vi "Configured Acquisition Trigger (Host)_20221229_Dual.vi"() -> ()   [LabVIEW 2021]
doc: "Use this VI as a template to design an application that acquires data using advanced triggering logic from the NI PXIe-5170R/5171R."
uses:
  Enums/Channel Numbers.ctl
  <vilib>/FPGAPlugInAG/PXIe-5172 (8CH - 410T)/niLvFpga_Open_PXIe-5172 (8CH - 410T).vi
  <vilib>/rvi/interface/common/dynamic/niFpgaDynamicAddResources.vi
  <vilib>/FPGAPlugInAG/Dynamic/niLvFpga_Close_Dynamic.vi
  <vilib>/rvi/interface/nirviOpenFPGA/nirviOpenFPGA.xnode
  FPGA Bitfiles/Multirecord Acquisition FPGA_20221228a_4.lvbitx
  <vilib>/rvi/interface/nirviCloseFPGA/nirviCloseFPGA.xnode
  Device Session/Device Session.lvclass
panel:
  out "Host Loop Count":i32
  out "Waveform Graph 1":T1(graph)
  out "TrigCfg Array":T2(array[cluster])
  out "TrigCount":u32[](array[numeric])
  in  "ResetTrig":bool=TRUE
  in  "Sliding Window Trigger":cluster{"Range":dbl, "StartCenter":dbl}[](array[cluster])=[{"Range"=2.01, "StartCenter"=0.0}, {"Range"=0.01, "StartCenter"=0.0}, {"Range"=5.0, "StartCenter"=0.0}, {"Range"=5.0, "StartCenter"=0.0}, {"Range"=5.0, "StartCenter"=0.0}, {"Range"=5.0, "StartCenter"=0.0}, {"Range"=5.0, "StartCenter"=0.0}, {"Range"=5.0, "StartCenter"=0.0}]
  out "actual sample rate":dbl format="%#_6p"
  in  "onboard sample clock rate":dbl(ring)=200000000.0 items=["250 MHz"=250000000.0, "200 MHz"=200000000.0, "150 MHz"=150000000.0]
  in  "impedance":enum8{"Default", "1 mega ohm", "50 ohm"}(ring)
  in  "vertical offset (V)":dbl format="%.2p"
  out "Waveform Graph 0":T1(graph)
  in  "mode":T3(ring)
  in  "decimation factor":u16=1
  in  "coupling":enum8{"Default", "DC", "AC"}(ring)
  in  "bandwidth":T4(ring)
  in  "pretrigger samples":u64=500
  in  "number of samples":u64=1000
  in  "RIO Device":tag="PXI2Slot3"
  in  "channel(s)":string="0,1,2,3,4,5,6,7"
  in  "vertical range (Vpp)":dbl=1.0 format="%.2p"
  out "error out":errorcluster
  in  "stop":bool
  # "RIO Device"
  # "Vertical Settings"
  # "Trigger Settings"
  # "Acquisition Settings"
  # "DSP"
  # "Clocking"
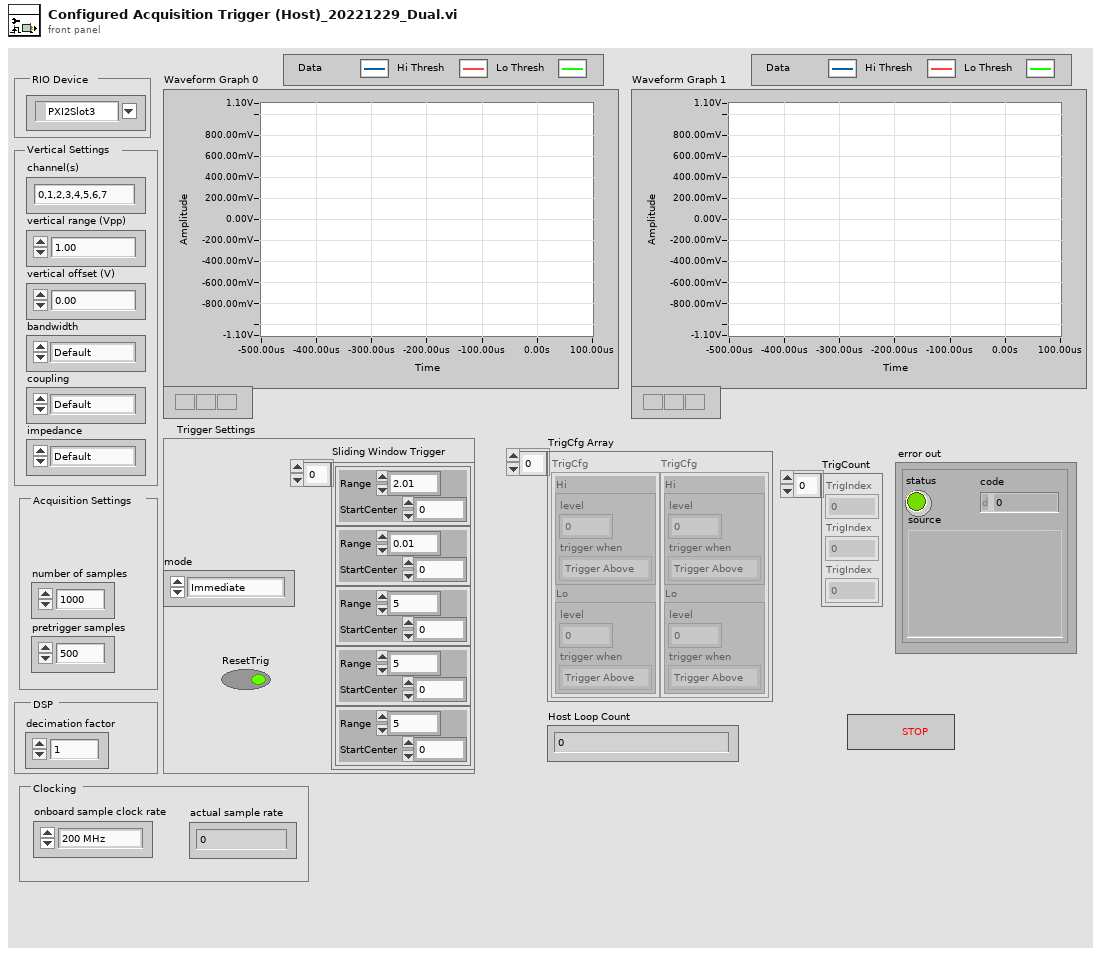
[diagram p1: front panel]
types:
  T1 = cluster{"relativeX":dbl, "sample rate":dbl, "data in":dbl[]}[]
  T2 = cluster{"Hi":cluster{"level":fxp<+/-,18,5>, "trigger when":enum8{"Trigger Above", "Trigger Below"}}, "Lo":cluster{"level":fxp<+/-,18,5>, "trigger when":enum8{"Trigger Above", "Trigger Below"}}}[]
  T3 = enum16{"Immediate", "A", "B", "OR", "AND", "A THEN B", "B THEN A", "High Resolution"}
  T4 = enum8{"Default", "Full Bandwidth", "Anti-alias Filter", "80 MHz FIR Filter", "40 MHz FIR Filter", "20 MHz FIR Filter"}
  T5 = typedef "Channel Numbers.ctl" = enum16{"0", "1", "2", "3", "4", "5", "6", "7"}
  T6 = typedef "niInstr Multirecord Acquisition v1 Host.lvclass/Scaling Coefficient.ctl" = cluster{"gain":dbl, "offset":dbl}
  T7 = typedef "ChannelWindowClust.ctl" = cluster{"HalfRange":fxp<+/-,18,5>, "StartCenter":fxp<+/-,18,5>}
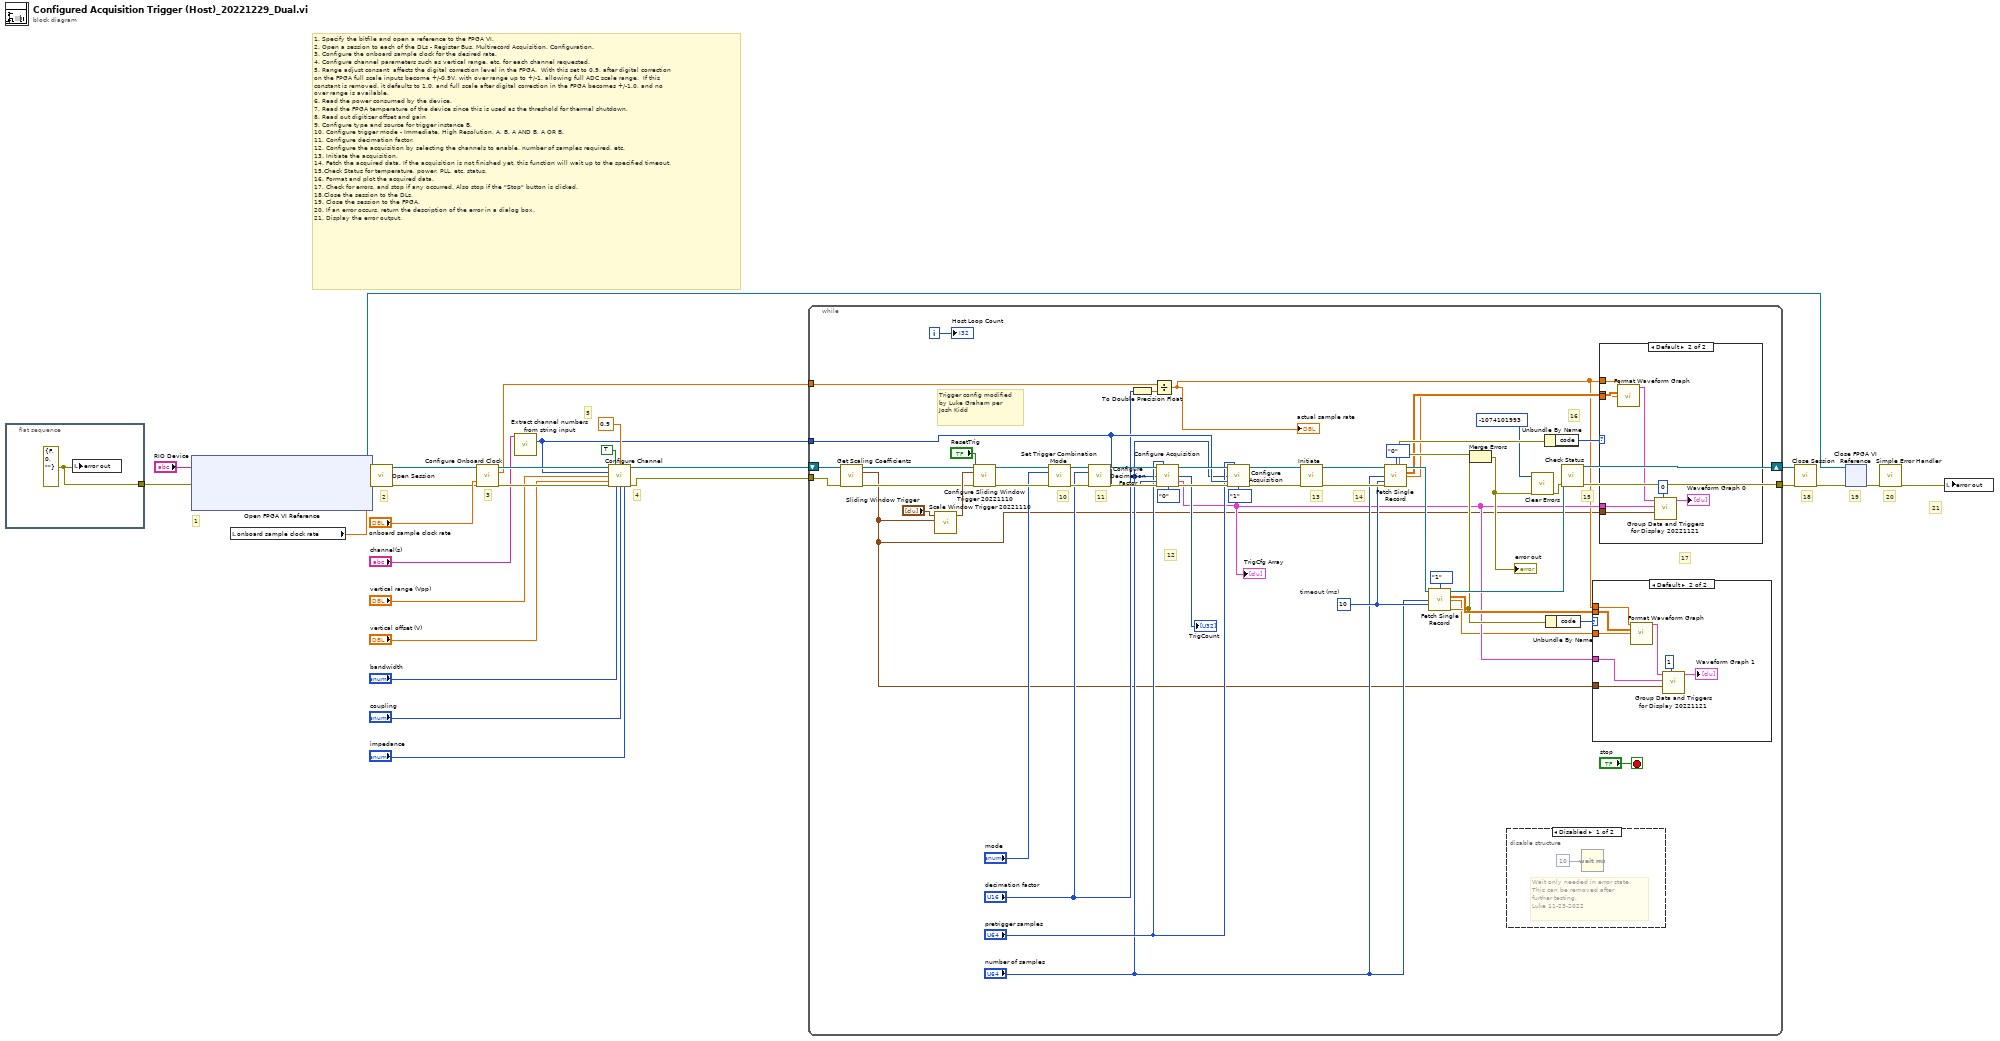
[diagram p0: block diagram]
diagram:
  # "4"
  # "5"
  # "3"
  # "21"
  # "20"
  # "19"
  # "18"
  # "1. Specify the bitfile and open a reference to the FPGA VI.\n2. Open a session to each of the DLs - Register Bus, Multirecord Acquisition, Configuration.\n3. Configure the onboard sample clock for the desired rate.\n4. Configure channel parameters such as vertical range, etc. for each channel requested.\n5. Range adjust consant  affects the digital correction level in the FPGA.  With this set to 0.9, after digital correction\non the FPGA full scale inputs become +/-0.9V, with over range up to +/-1, allowing full ADC scale range.  If this \nconstant is removed, it defaults to 1.0, and full scale after digital correction in the FPGA becomes +/-1.0, and no\nover range is available.  \n6. Read the power consumed by the device.\n7. Read the FPGA temperature of the device since this is used as the threshold for thermal shutdown.\n8. Read out digitizer offset and gain\n9. Configure type and source for trigger instance B.\n10. Configure trigger mode - Immediate, High Resolution, A, B, A AND B, A OR B.\n11. Configure decimation factor.\n12. Configure the acquisition by selecting the channels to enable, number of samples required, etc.\n13. Initiate the acquisition.\n14. Fetch the acquired data. If the acquisition is not finished yet, this function will wait up to the specified timeout.\n15.Check Status for temperature, power, PLL, etc. status. \n16. Format and plot the acquired data.\n17. Check for errors, and stop if any occurred. Also stop if the \"Stop\" button is clicked.\n18.Close the session to the DLs.\n19. Close the session to the FPGA.\n20. If an error occurs, return the description of the error in a dialog box.\n21. Display the error output."
  # "2"
  # "1"
  n1 = flat-sequence {
    tunnel: [w28] -> w19
    frame #0 {
      w28 = errorcluster {"status"=FALSE, "code"=0, "source"=""} ("error constant")
      n2 = local write "error out"(w28) -> ()
    }
  }
  n3 = xnode "Open FPGA VI Reference"("error in"=w19, "resource name"="RIO Device") -> ("FPGA VI Reference Out"=w23:refnum<k20>, "error out"=w18:errorcluster)
  n4 = local read "onboard sample clock rate"() -> (w21:dbl)
  n5 = call "Open Session.vi"("FPGA VI Ref"=w23, "adc clock rate (Hz)"=w21, "error in"=w18) -> ("device session out"=w8:refnum<class "Device Session.lvclass">, "error out"=w7:errorcluster)  [unwired: 11 in]
  n6 = call "Configure Onboard Clock.vi"("device session in"=w8, "adc clock rate (Hz)"="onboard sample clock rate", "error in"=w7) -> ("device session out"=w17:refnum<class "Device Session.lvclass">, "actual adc clock rate (Hz)"=w3:dbl, "error out"=w12:errorcluster)  [unwired: 9 in, 1 out]
  n7 = call "Extract channel numbers from string input.vi"("channel input"="channel(s)") -> ("array of chans"=w4:u32[])  [unwired: 13 in, 1 out]
  n8 = call "Configure Channel.vi"("device session in"=w17, "enable channel (T)"=TRUE ("enable channel"), "range adjust"=0.9, "channels"=w4, "vertical range (Vpp)"="vertical range (Vpp)", "vertical offset (V)"="vertical offset (V)", "error in"=w12, "bandwidth"="bandwidth", "coupling"="coupling", "impedance"="impedance") -> ("device session out"=w1:refnum<class "Device Session.lvclass">, "error out"=w2:errorcluster)  [unwired: 4 in]
  n9 = while {
    shift-right: [w72] -> w26
    shift-left: w1 -> [w31]
    tunnel: [w68] -> w27
    tunnel: w4 -> [w46]
    tunnel: w3 -> [w47]
    tunnel: w2 -> [w33]
    i -> [w36]
    stop <- "stop" stop-if-true
    w64 = 10  # timeout (ms)
    # "Trigger config modified by Luke Graham per Josh Kidd"
    # "15"
    # "11"
    # "17"
    # "16"
    # "10"
    # "14"
    # "13"
    # "12"
    n10 = call "Get Scaling Coefficients.vi"("device session in"=w31, "error in"=w33) -> ("device session out"=w30:refnum<class "Device Session.lvclass">, "scaling coefficients"=w29:T6[], "error out"=w32:errorcluster)  [unwired: 11 in]
    n11 = call "Scale Window Trigger 20221110.vi"("scaling coefficients"=w29, "Sliding Window Trigger"="Sliding Window Trigger") -> ("Sliding Window Trigger (FXP)"=w34:T7[])  [unwired: 9 in]
    n12 = call "Configure Sliding Window Trigger 20221110.vi"("device session in"=w30, "Sliding Window Triggers (FXP)"=w34, "ResetTrig"="ResetTrig", "error in"=w32) -> ("device session out"=w71:refnum<class "Device Session.lvclass">, "error out"=w70:errorcluster)  [unwired: 10 in]
    n13 = call "Set Trigger Combination Mode.vi"("device session in"=w71, "mode"="mode", "error in"=w70) -> ("device session out"=w76:refnum<class "Device Session.lvclass">, "error out"=w75:errorcluster)  [unwired: 11 in]
    n14 = call "Configure Decimation Factor.vi"("device session in"=w76, "decimation factor"="decimation factor", "error in"=w75) -> ("device session out"=w73:refnum<class "Device Session.lvclass">, "error out"=w74:errorcluster)  [unwired: 11 in]
    n15 = To Double Precision Float(number="decimation factor") -> (double precision float=w77:dbl)
    n16 = Divide(x=w47, y=w77) -> (x/y=w37:dbl)
    "actual sample rate" <- w37
    n17 = call "Configure Acquisition.vi"("device session in"=w73, "pretrigger samples"="pretrigger samples", "number of samples"="number of samples", "channels to store"=w46, "error in"=w74, "Chan#"=Channel_Numbers."0") -> ("device session out"=w62:refnum<class "Device Session.lvclass">, "TrigCount"=→"TrigCount":u32[], "TrigCfg Array"=w39:T2, "error out"=w59:errorcluster)  [unwired: 5 in, 1 out]
    "TrigCfg Array" <- w39
    n18 = call "Configure Acquisition.vi"("device session in"=w62, "pretrigger samples"="pretrigger samples", "number of samples"="number of samples", "channels to store"=w46, "error in"=w59, "Chan#"=Channel_Numbers."1") -> ("device session out"=w61:refnum<class "Device Session.lvclass">, "error out"=w60:errorcluster)  [unwired: 5 in, 3 out]
    n19 = call "Initiate.vi"("device session in"=w61, "error in"=w60) -> ("device session out"=w79:refnum<class "Device Session.lvclass">, "error out"=w80:errorcluster)  [unwired: 12 in]
    n20 = call "Fetch Single Record.vi"("device session in"=w79, "number of samples"="number of samples", "timeout (ms)"=w64, "error in"=w80, "Chan#"=Channel_Numbers."0") -> ("device session out"=w66:refnum<class "Device Session.lvclass">, "data"=w41:dbl[][], "relativeX (samples)"=w40:dbl, "error out"=w54:errorcluster)  [unwired: 6 in, 1 out]
    n21 = call "Fetch Single Record.vi"("device session in"=w66, "number of samples"="number of samples", "timeout (ms)"=w64, "Chan#"=Channel_Numbers."1") -> ("device session out"=w65:refnum<class "Device Session.lvclass">, "data"=w63:dbl[][], "relativeX (samples)"=w38:dbl, "error out"=w49:errorcluster)  [unwired: 7 in, 1 out]
    n22 = Merge Errors(w54, w49) -> (w53:errorcluster)
    "error out" <- w53
    n23 = disable-structure shown="Disabled" {
      frame Disabled {
        # "Wait only needed in error state.\nThis can be removed after\nfurther testing.\nLuke 11-23-2022"
        n24 = Wait (ms)(milliseconds to wait=u32 10) -> ()  [unwired: 1 out]
      }
      frame Enabled {
      }
    }
    n25 = call <vilib>:"Clear Errors.vi"("error in (no error)"=w53, "specific error code to clear (0: all)"=-1074101993) -> ("error out"=w52:errorcluster)  [unwired: 4 in, 1 out]
    n26 = Unbundle By Name(w54) -> ("code"=w55:i32)
    n27 = Unbundle By Name(w49) -> ("code"=w50:i32)
    n28 = call "Check Status.vi"("device session in"=w65, "error in"=w52) -> ("device session out"=w72:refnum<class "Device Session.lvclass">, "error out"=w68:errorcluster)  [unwired: 12 in]
    n29 = case shown="Default" w50 {
      tunnel: w63 -> [_ w88]
      tunnel: w39 -> [_ w89]
      tunnel: w29 -> [_ w85]
      tunnel: w38 -> [_ w83]
      tunnel: w37 -> [_ w82]
      frame -1074101998, -1074101995, -1074101993 {
      }
      frame Default {
        n30 = call "Format Waveform Graph.vi"("sample rate (Hz)"=w82, "data in"=w88, "relativeX (samples)"=w83) -> ("waveform out"=w87:T1)  [unwired: 12 in]
        n31 = call "Group Data and Triggers for Display 20221121.vi"("Chan"=1, "scaling coefficients"=w85, "TrigCfg"=w89, "Data waveform"=w87) -> ("Data for Display"=→"Waveform Graph 1":T1)  [unwired: 7 in]
      }
    }
    n32 = case shown="Default" w55 {
      tunnel: w39 -> [_ w95]
      tunnel: w29 -> [_ w96]
      tunnel: w37 -> [_ w94]
      tunnel: w41 -> [_ w93]
      tunnel: w40 -> [_ w92]
      frame -1074101998, -1074101995, -1074101993 {
      }
      frame Default {
        n33 = call "Format Waveform Graph.vi"("sample rate (Hz)"=w94, "data in"=w93, "relativeX (samples)"=w92) -> ("waveform out"=w91:T1)  [unwired: 12 in]
        n34 = call "Group Data and Triggers for Display 20221121.vi"("Chan"=0, "scaling coefficients"=w96, "TrigCfg"=w95, "Data waveform"=w91) -> ("Data for Display"=→"Waveform Graph 0":T1)  [unwired: 7 in]
      }
    }
    "Host Loop Count" <- w36
  }
  n35 = call "Close Session.vi"("device session in"=w26, "error in"=w27) -> ("error out"=w24:errorcluster)  [unwired: 13 in]
  n36 = xnode "Close FPGA VI Reference"("FPGA VI Reference In"=w23, "error in"=w24) -> ("error out"=w22:errorcluster)
  n37 = call <vilib>:"Simple Error Handler.vi"("error in (no error)"=w22) -> ("error out"=w20:errorcluster)  [unwired: 4 in, 4 out]
  n38 = local write "error out"(w20) -> ()
